vi "UHR-Fleezers Control (host) - 12.4.vi"() -> ()   [LabVIEW 2012] (continued)
                                tunnel: w627 -> [w628]
                                frame #0 {
                                n357 = property on="Trap Pos FB SP" class="DigNum (strict)"("Val(Sgnl)"=w628) -> ()  [unwired: 2 in, 2 out]
                                }
                                frame #1 {
                                n358 = Wait (ms)(milliseconds to wait=u32 700) -> ()  [unwired: 1 out]
                                }
                                frame #2 {
                                n359 = local read "Action (%)"() -> (w633:dbl)
                                n360 = Absolute Value(x=w633) -> (abs(x)=w632:dbl)
                                n361 = Greater?(x=w632, y=70.0) -> (0:w630:bool)
                                n362 = property on="Remove Action Offset" class="Bool (strict)"("Val(Sgnl)"=w630) -> ()  [unwired: 2 in, 2 out]
                                }
                                frame #3 {
                                n363 = for {
                                N: 4 -> [_]
                                n364 = flat-sequence {
                                frame #0 {
                                n365 = Wait (ms)(milliseconds to wait=u32 500) -> ()  [unwired: 1 out]
                                }
                                frame #1 {
                                n366 = local read "Action (%)"() -> (w639:dbl)
                                n367 = Absolute Value(x=w639) -> (abs(x)=w638:dbl)
                                n368 = Greater?(x=w638, y=70.0) -> (0:w636:bool)
                                n369 = property on="Remove Action Offset" class="Bool (strict)"("Val(Sgnl)"=w636) -> ()  [unwired: 2 in, 2 out]
                                }
                                }
                                }
                                }
                                frame #4 {
                                n370 = Wait (ms)(milliseconds to wait=u32 500) -> ()  [unwired: 1 out]
                                }
                                frame #5 {
                                n371 = local read "Mean"() -> (w647:dbl)
                                n372 = Greater?(x=w647, y=11.0) -> (0:w641:bool)
                                n373 = Not(x=w641) -> (.not. x?=w642:bool)
                                n374 = And(x=w642, y="Shift confocal") -> (x .and. y?=w644:bool)
                                n375 = And(x=w641, y="Shift confocal") -> (x .and. y?=w645:bool)
                                n376 = case shown="True" w645 {
                                frame False {
                                }
                                frame True {
                                n377 = local read "Confocal Y 2 (V)"() -> (w651:dbl)
                                n378 = local read "Confocal X 2 (V)"() -> (w650:dbl)
                                n379 = property on="AO1" class="Slide (strict)"("Val(Sgnl)"=w651) -> ()  [unwired: 2 in, 2 out]
                                n380 = property on="AO2" class="Slide (strict)"("Val(Sgnl)"=w650) -> ()  [unwired: 2 in, 2 out]
                                }
                                }
                                n381 = case shown="True" w644 {
                                frame False {
                                }
                                frame True {
                                n382 = local read "Confocal Y 1 (V)"() -> (w649:dbl)
                                n383 = local read "Confocal X 1 (V)"() -> (w648:dbl)
                                n384 = property on="AO1" class="Slide (strict)"("Val(Sgnl)"=w649) -> ()  [unwired: 2 in, 2 out]
                                n385 = property on="AO2" class="Slide (strict)"("Val(Sgnl)"=w648) -> ()  [unwired: 2 in, 2 out]
                                }
                                }
                                }
                                frame #6 {
                                n386 = Wait (ms)(milliseconds to wait=u32 1500) -> ()  [unwired: 1 out]
                                }
                                frame #7 {
                                n387 = property on="Rem fb disp offset" class="Bool (strict)"("Val(Sgnl)"=TRUE ("Value (Signaling)")) -> ()  [unwired: 2 in, 2 out]
                                }
                                }
                                }
                                frame True {
                                n388 = flat-sequence {
                                tunnel: w654 -> [w655]
                                frame #0 {
                                n389 = property on="Trap Delta (MHz)" class="DigNum (strict)"("Val(Sgnl)"=w655) -> ()  [unwired: 2 in, 2 out]
                                }
                                frame #1 {
                                n390 = Wait (ms)(milliseconds to wait=u32 500) -> ()  [unwired: 1 out]
                                }
                                frame #2 {
                                n391 = local read "Shift confocal"() -> (w661:bool)
                                n392 = local read "Mean"() -> (w663:dbl)
                                n393 = Greater?(x=w663, y=11.0) -> (0:w660:bool)
                                n394 = Not(x=w660) -> (.not. x?=w659:bool)
                                n395 = And(x=w659, y=w661) -> (x .and. y?=w657:bool)
                                n396 = And(x=w660, y=w661) -> (x .and. y?=w658:bool)
                                n397 = case shown="True" w658 {
                                frame False {
                                }
                                frame True {
                                n398 = local read "Confocal Y 2 (V)"() -> (w667:dbl)
                                n399 = local read "Confocal X 2 (V)"() -> (w666:dbl)
                                n400 = property on="AO2" class="Slide (strict)"("Val(Sgnl)"=w666) -> ()  [unwired: 2 in, 2 out]
                                n401 = property on="AO1" class="Slide (strict)"("Val(Sgnl)"=w667) -> ()  [unwired: 2 in, 2 out]
                                }
                                }
                                n402 = case shown="True" w657 {
                                frame False {
                                }
                                frame True {
                                n403 = local read "Confocal X 1 (V)"() -> (w664:dbl)
                                n404 = local read "Confocal Y 1 (V)"() -> (w665:dbl)
                                n405 = property on="AO2" class="Slide (strict)"("Val(Sgnl)"=w664) -> ()  [unwired: 2 in, 2 out]
                                n406 = property on="AO1" class="Slide (strict)"("Val(Sgnl)"=w665) -> ()  [unwired: 2 in, 2 out]
                                }
                                }
                                }
                                }
                                }
                                }
                                }
                                }
                                }
                                frame "Image" {
                                n407 = property on="Confocal Image" class="Bool (strict)"("Val(Sgnl)"=TRUE ("Value (Signaling)")) -> ()  [unwired: 2 in, 2 out]
                                }
                              }
                              n408 = local write "Fl. High"(FALSE ("Fl. High")) -> ()
                              n409 = local read "Time (s)"() -> (w601:dbl)
                            }
                            frame #1 {
                              n410 = case shown="True" "Auto F Reset" {
                                tunnel: w673 -> [_ w678]
                                tunnel: w672 -> [_ w677]
                                tunnel: w671 -> [_ w676]
                                tunnel: w670 -> [_ w675]
                                frame False {
                                }
                                frame True {
                                n411 = node-c288() -> (w680:T22)  [unwired: 4 in]
                                n412 = timed-loop {
                                timing: w680 -> [_]
                                timing-out: [_] -> w679
                                tunnel: w678 -> [w685]
                                tunnel: w677 -> [w684]
                                tunnel: w676 -> [w683]
                                tunnel: w675 -> [w682]
                                stop <- w681 stop-if-true
                                n413 = node-c288() -> ()  [unwired: 1 in, 1 out]
                                n414 = local read "Fl. Delta Thresh. (kHz)"() -> (w694:dbl)
                                n415 = local read "APD to Watch"() -> (w695:bool)
                                n416 = local read "Delta Fl. 1"() -> (w696:dbl)
                                n417 = local read "Delta Fl. 2"() -> (w697:dbl)
                                n418 = local read "Fl. Triggered..."() -> (w688:bool)
                                n419 = local read "Stop All"() -> (w689:bool)
                                n420 = local read "Reset Force"() -> (w687:bool)
                                n421 = Multiply(x=w694, y=1000.0) -> (x*y=w692:dbl)
                                n422 = Select(t=w696, s=w695, f=w697) -> (s? t:f=w691:dbl)
                                n423 = Not(x=w688) -> (.not. x?=w686:bool)
                                n424 = Greater?(x=w691, y=w692) -> (0:w690:bool)
                                n425 = Compound Arithmetic op=OR(w690, w689, w686, w687) -> (w681:bool)
                                n426 = case shown="True" w681 {
                                tunnel: w685 -> [_ w701]
                                tunnel: w684 -> [_ w705]
                                tunnel: w683 -> [_ w704]
                                tunnel: w682 -> [_ w703]
                                frame False {
                                }
                                frame True {
                                n427 = case shown="\"Yank\"" w705 {
                                tunnel: w704 -> [_ w715]
                                tunnel: w703 -> [_ w713]
                                frame "Image", Default {
                                }
                                frame "Yank" {
                                n428 = flat-sequence {
                                tunnel: [w718] -> w716
                                tunnel: w715 -> [w718]
                                tunnel: [w717] -> w714
                                tunnel: w713 -> [w717]
                                tunnel: w716 -> [w724]
                                tunnel: w714 -> [w722]
                                frame #0 {
                                n429 = local read "Yank Delay (s)"() -> (w721:dbl)
                                n430 = Multiply(x=w721, y=1000.0) -> (x*y=w719:dbl)
                                n431 = Wait (ms)(milliseconds to wait=w719) -> ()  [unwired: 1 out]
                                }
                                frame #1 {
                                n432 = local read "Yank to which?"() -> (w723:bool)
                                n433 = case shown="False" w723 {
                                tunnel: w724 -> [_ w752]
                                tunnel: w722 -> [w725 _]
                                frame False {
                                n434 = flat-sequence {
                                tunnel: w725 -> [w726]
                                frame #0 {
                                n435 = property on="Trap Pos FB SP" class="DigNum (strict)"("Val(Sgnl)"=w726) -> ()  [unwired: 2 in, 2 out]
                                }
                                frame #1 {
                                n436 = Wait (ms)(milliseconds to wait=u32 700) -> ()  [unwired: 1 out]
                                }
                                frame #2 {
                                n437 = local read "Action (%)"() -> (w731:dbl)
                                n438 = Absolute Value(x=w731) -> (abs(x)=w730:dbl)
                                n439 = Greater?(x=w730, y=70.0) -> (0:w728:bool)
                                n440 = property on="Remove Action Offset" class="Bool (strict)"("Val(Sgnl)"=w728) -> ()  [unwired: 2 in, 2 out]
                                }
                                frame #3 {
                                n441 = for {
                                N: 4 -> [_]
                                n442 = flat-sequence {
                                frame #0 {
                                n443 = Wait (ms)(milliseconds to wait=u32 500) -> ()  [unwired: 1 out]
                                }
                                frame #1 {
                                n444 = local read "Action (%)"() -> (w737:dbl)
                                n445 = Absolute Value(x=w737) -> (abs(x)=w736:dbl)
                                n446 = Greater?(x=w736, y=70.0) -> (0:w734:bool)
                                n447 = property on="Remove Action Offset" class="Bool (strict)"("Val(Sgnl)"=w734) -> ()  [unwired: 2 in, 2 out]
                                }
                                }
                                }
                                }
                                frame #4 {
                                n448 = Wait (ms)(milliseconds to wait=u32 500) -> ()  [unwired: 1 out]
                                }
                                frame #5 {
                                n449 = local read "Shift confocal"() -> (w742:bool)
                                n450 = local read "Mean"() -> (w745:dbl)
                                n451 = Greater?(x=w745, y=11.0) -> (0:w741:bool)
                                n452 = Not(x=w741) -> (.not. x?=w740:bool)
                                n453 = And(x=w741, y=w742) -> (x .and. y?=w743:bool)
                                n454 = And(x=w740, y=w742) -> (x .and. y?=w739:bool)
                                n455 = case shown="True" w743 {
                                frame False {
                                }
                                frame True {
                                n456 = local read "Confocal X 2 (V)"() -> (w748:dbl)
                                n457 = local read "Confocal Y 2 (V)"() -> (w749:dbl)
                                n458 = property on="AO2" class="Slide (strict)"("Val(Sgnl)"=w748) -> ()  [unwired: 2 in, 2 out]
                                n459 = property on="AO1" class="Slide (strict)"("Val(Sgnl)"=w749) -> ()  [unwired: 2 in, 2 out]
                                }
                                }
                                n460 = case shown="True" w739 {
                                frame False {
                                }
                                frame True {
                                n461 = local read "Confocal Y 1 (V)"() -> (w747:dbl)
                                n462 = local read "Confocal X 1 (V)"() -> (w746:dbl)
                                n463 = property on="AO1" class="Slide (strict)"("Val(Sgnl)"=w747) -> ()  [unwired: 2 in, 2 out]
                                n464 = property on="AO2" class="Slide (strict)"("Val(Sgnl)"=w746) -> ()  [unwired: 2 in, 2 out]
                                }
                                }
                                }
                                frame #6 {
                                n465 = Wait (ms)(milliseconds to wait=u32 1500) -> ()  [unwired: 1 out]
                                }
                                frame #7 {
                                n466 = property on="Rem fb disp offset" class="Bool (strict)"("Val(Sgnl)"=TRUE ("Value (Signaling)")) -> ()  [unwired: 2 in, 2 out]
                                }
                                }
                                }
                                frame True {
                                n467 = flat-sequence {
                                tunnel: w752 -> [w753]
                                frame #0 {
                                n468 = property on="Trap Delta (MHz)" class="DigNum (strict)"("Val(Sgnl)"=w753) -> ()  [unwired: 2 in, 2 out]
                                }
                                frame #1 {
                                n469 = Wait (ms)(milliseconds to wait=u32 500) -> ()  [unwired: 1 out]
                                }
                                frame #2 {
                                n470 = local read "Shift confocal"() -> (w759:bool)
                                n471 = local read "Mean"() -> (w760:dbl)
                                n472 = Greater?(x=w760, y=11.0) -> (0:w758:bool)
                                n473 = And(x=w758, y=w759) -> (x .and. y?=w756:bool)
                                n474 = Not(x=w758) -> (.not. x?=w757:bool)
                                n475 = And(x=w757, y=w759) -> (x .and. y?=w755:bool)
                                n476 = case shown="True" w756 {
                                frame False {
                                }
                                frame True {
                                n477 = local read "Confocal Y 2 (V)"() -> (w765:dbl)
                                n478 = local read "Confocal X 2 (V)"() -> (w764:dbl)
                                n479 = property on="AO1" class="Slide (strict)"("Val(Sgnl)"=w765) -> ()  [unwired: 2 in, 2 out]
                                n480 = property on="AO2" class="Slide (strict)"("Val(Sgnl)"=w764) -> ()  [unwired: 2 in, 2 out]
                                }
                                }
                                n481 = case shown="True" w755 {
                                frame False {
                                }
                                frame True {
                                n482 = local read "Confocal Y 1 (V)"() -> (w763:dbl)
                                n483 = local read "Confocal X 1 (V)"() -> (w762:dbl)
                                n484 = property on="AO2" class="Slide (strict)"("Val(Sgnl)"=w762) -> ()  [unwired: 2 in, 2 out]
                                n485 = property on="AO1" class="Slide (strict)"("Val(Sgnl)"=w763) -> ()  [unwired: 2 in, 2 out]
                                }
                                }
                                }
                                }
                                }
                                }
                                }
                                }
                                }
                                }
                                n486 = local read "Time (s)"() -> (w700:dbl)
                                n487 = Subtract(x=w701, y=w700) -> (x-y=w712:dbl)
                                n488 = Number To Decimal String(number=w712, width (-)=i16 0) -> (decimal integer string=w710:string)
                                n489 = Concatenate Strings(w710, " s fluorescence event") -> (w707:string)
                                n490 = local read "Messages"() -> (w708:string)
                                n491 = local write "Duration (s)"(w712) -> ()
                                n492 = call "Update messages.vi"("Message to add"=w707, "Old message string"=w708) -> ("New message string"=w706:string)
                                n493 = local write "Messages"(w706) -> ()
                                n494 = call <vilib>:"Beep.vi"() -> ()  [unwired: 12 in]
                                n495 = local write "Reset Force"(FALSE ("Force Reset")) -> ()
                                n496 = local write "Fl. High"(TRUE ("Fl. High")) -> ()
                                n497 = local write "Waiting"(TRUE ("Waiting")) -> ()
                                }
                                }
                                n498 = node-c288() -> ()  [unwired: 1 in, 1 out]
                                }
                                n499 = node-c288(w679) -> ()  [unwired: 1 out]
                                }
                              }
                            }
                          }
                          n500 = local read "Trap Delta (MHz)"() -> (w591:dbl)
                          n501 = local read "Trap Pos FB SP"() -> (w589:fxp<+/-,16,1>)
                        }
                      }
                    }
                    frame True {
                      n502 = flat-sequence {
                        tunnel: w776 -> [w786]
                        tunnel: [w786] -> w780
                        tunnel: w779 -> [w785]
                        tunnel: [w785] -> w778
                        tunnel: [w784] -> w777
                        tunnel: w775 -> [w783]
                        tunnel: [w782] -> w774
                        tunnel: w771 -> [w781]
                        tunnel: [w781] -> w770
                        tunnel: w780 -> [w856]
                        tunnel: w778 -> [w855]
                        tunnel: w777 -> [w854]
                        tunnel: w774 -> [w853]
                        tunnel: w770 -> [w852]
                        tunnel: [w853] -> w773
                        frame #0 {
                          n503 = call <vilib>:"Beep.vi"() -> ()  [unwired: 3 in, 9 out]
                          n504 = local write "Waiting"(FALSE ("Waiting")) -> ()
                          n505 = Increment(x=w783) -> (x+1=w782:u8)
                          n506 = case shown="\"Yank\"" w785 {
                            tunnel: w782 -> [_ _ w792]
                            frame "Image" {
                              n507 = property on="Confocal Image" class="Bool (strict)"("Val(Sgnl)"=TRUE ("Value (Signaling)")) -> ()  [unwired: 2 in, 2 out]
                            }
                            frame "Alarm", Default {
                            }
                            frame "Yank" {
                              n508 = flat-sequence {
                                tunnel: w792 -> [w795]
                                tunnel: [w794] -> w791
                                tunnel: ["N Array El"] -> w790
                                tunnel: w791 -> [w809]
                                tunnel: w790 -> [w805]
                                frame #0 {
                                n509 = Multiply(x="Yank Delay (s)", y=1000.0) -> (x*y=w798:dbl)
                                n510 = Quotient & Remainder(x=w795, y="N Array El") -> (x-y*floor(x/y)=w794:u8)  [unwired: 1 out]
                                n511 = Wait (ms)(milliseconds to wait=w798) -> ()  [unwired: 1 out]
                                }
                                frame #1 {
                                n512 = Random Number (0-1)() -> (number: 0 to 1=w806:dbl)
                                n513 = Multiply(x=w805, y=w806) -> (x*y=w804:dbl)
                                n514 = Round Toward -Infinity(1:w804) -> (0:w803:dbl)
                                n515 = Select(t=w803, s="Random Choice", f=w809) -> (s? t:f=w807:dbl)
                                n516 = Select(t="Yank to Trap Delta (MHz)", s="Yank to which?", f="Yank to SP") -> (s? t:f=w800:dbl[])
                                n517 = Index Array(array=w800, index=w807) -> (element=w810:dbl)
                                n518 = case shown="False" "Yank to which?" {
                                tunnel: w810 -> [w811 w837]
                                frame False {
                                n519 = flat-sequence {
                                tunnel: w811 -> [w812]
                                frame #0 {
                                n520 = property on="Trap Pos FB SP" class="DigNum (strict)"("Val(Sgnl)"=w812) -> ()  [unwired: 2 in, 2 out]
                                }
                                frame #1 {
                                n521 = Wait (ms)(milliseconds to wait=u32 700) -> ()  [unwired: 1 out]
                                }
                                frame #2 {
                                n522 = local read "Action (%)"() -> (w817:dbl)
                                n523 = Absolute Value(x=w817) -> (abs(x)=w816:dbl)
                                n524 = Greater?(x=w816, y=70.0) -> (0:w814:bool)
                                n525 = property on="Remove Action Offset" class="Bool (strict)"("Val(Sgnl)"=w814) -> ()  [unwired: 2 in, 2 out]
                                }
                                frame #3 {
                                n526 = for {
                                N: 4 -> [_]
                                n527 = flat-sequence {
                                frame #0 {
                                n528 = Wait (ms)(milliseconds to wait=u32 500) -> ()  [unwired: 1 out]
                                }
                                frame #1 {
                                n529 = local read "Action (%)"() -> (w823:dbl)
                                n530 = Absolute Value(x=w823) -> (abs(x)=w822:dbl)
                                n531 = Greater?(x=w822, y=70.0) -> (0:w820:bool)
                                n532 = property on="Remove Action Offset" class="Bool (strict)"("Val(Sgnl)"=w820) -> ()  [unwired: 2 in, 2 out]
                                }
                                }
                                }
                                }
                                frame #4 {
                                n533 = local read "Shift confocal"() -> (w827:bool)
                                n534 = local read "Mean"() -> (w830:dbl)
                                n535 = Greater?(x=w830, y=11.0) -> (0:w826:bool)
                                n536 = Not(x=w826) -> (.not. x?=w825:bool)
                                n537 = And(x=w825, y=w827) -> (x .and. y?=w824:bool)
                                n538 = And(x=w826, y=w827) -> (x .and. y?=w828:bool)
                                n539 = case shown="True" w828 {
                                frame False {
                                }
                                frame True {
                                n540 = local read "Confocal X 2 (V)"() -> (w833:dbl)
                                n541 = local read "Confocal Y 2 (V)"() -> (w834:dbl)
                                n542 = property on="AO2" class="Slide (strict)"("Val(Sgnl)"=w833) -> ()  [unwired: 2 in, 2 out]
                                n543 = property on="AO1" class="Slide (strict)"("Val(Sgnl)"=w834) -> ()  [unwired: 2 in, 2 out]
                                }
                                }
                                n544 = case shown="True" w824 {
                                frame False {
                                }
                                frame True {
                                n545 = local read "Confocal X 1 (V)"() -> (w831:dbl)
                                n546 = local read "Confocal Y 1 (V)"() -> (w832:dbl)
                                n547 = property on="AO1" class="Slide (strict)"("Val(Sgnl)"=w832) -> ()  [unwired: 2 in, 2 out]
                                n548 = property on="AO2" class="Slide (strict)"("Val(Sgnl)"=w831) -> ()  [unwired: 2 in, 2 out]
                                }
                                }
                                }
                                frame #5 {
                                n549 = Wait (ms)(milliseconds to wait=u32 1500) -> ()  [unwired: 1 out]
                                }
                                frame #6 {
                                n550 = property on="Rem fb disp offset" class="Bool (strict)"("Val(Sgnl)"=TRUE ("Value (Signaling)")) -> ()  [unwired: 2 in, 2 out]
                                }
                                }
                                }
                                frame True {
                                n551 = flat-sequence {
                                tunnel: w837 -> [w838]
                                frame #0 {
                                n552 = property on="Trap Delta (MHz)" class="DigNum (strict)"("Val(Sgnl)"=w838) -> ()  [unwired: 2 in, 2 out]
                                }
                                frame #1 {
                                n553 = Wait (ms)(milliseconds to wait=u32 500) -> ()  [unwired: 1 out]
                                }
                                frame #2 {
                                n554 = local read "Shift confocal"() -> (w842:bool)
                                n555 = local read "Mean"() -> (w840:dbl)
                                n556 = Greater?(x=w840, y=11.0) -> (0:w843:bool)
                                n557 = Not(x=w843) -> (.not. x?=w844:bool)
                                n558 = And(x=w844, y=w842) -> (x .and. y?=w846:bool)
                                n559 = And(x=w843, y=w842) -> (x .and. y?=w845:bool)
                                n560 = case shown="True" w845 {
                                frame False {
                                }
                                frame True {
                                n561 = local read "Confocal Y 2 (V)"() -> (w850:dbl)
                                n562 = local read "Confocal X 2 (V)"() -> (w849:dbl)
                                n563 = property on="AO1" class="Slide (strict)"("Val(Sgnl)"=w850) -> ()  [unwired: 2 in, 2 out]
                                n564 = property on="AO2" class="Slide (strict)"("Val(Sgnl)"=w849) -> ()  [unwired: 2 in, 2 out]
                                }
                                }
                                n565 = case shown="True" w846 {
                                frame False {
                                }
                                frame True {
                                n566 = local read "Confocal X 1 (V)"() -> (w847:dbl)
                                n567 = local read "Confocal Y 1 (V)"() -> (w848:dbl)
                                n568 = property on="AO2" class="Slide (strict)"("Val(Sgnl)"=w847) -> ()  [unwired: 2 in, 2 out]
                                n569 = property on="AO1" class="Slide (strict)"("Val(Sgnl)"=w848) -> ()  [unwired: 2 in, 2 out]
                                }
                                }
                                }
                                }
                                }
                                }
                                }
                              }
                            }
                          }
                          n570 = local read "Time (s)"() -> (w784:dbl)
                          "Fl. High" <- TRUE ("Yanking")
                        }
                        frame #1 {
                          n571 = local read "Auto F Reset"() -> (w851:bool)
                          n572 = case shown="True" w851 {
                            tunnel: w856 -> [_ w860]
                            tunnel: w855 -> [_ w859]
                            tunnel: w854 -> [_ w858]
                            tunnel: w852 -> [_ w857]
                            frame False {
                            }
                            frame True {
                              n573 = node-c288() -> (w862:T22)  [unwired: 4 out]
                              n574 = timed-loop {
                                timing: w862 -> [_]
                                timing-out: [_] -> w861
                                tunnel: w860 -> [w880]
                                tunnel: w859 -> [w879]
                                tunnel: w858 -> [w878]
                                tunnel: w857 -> [w877]
                                stop <- w863 stop-if-true
                                n575 = node-c288() -> ()  [unwired: 2 out]
                                n576 = local read "Fl. Delta Thresh. (kHz)"() -> (w871:dbl)
                                n577 = local read "Fl. Triggered..."() -> (w876:bool)
                                n578 = local read "Delta Fl. 1"() -> (w867:dbl)
                                n579 = local read "Delta Fl. 2"() -> (w865:dbl)
                                n580 = local read "Stop All"() -> (w874:bool)
                                n581 = local read "APD to Watch"() -> (w866:bool)
                                n582 = Select(t=w867, s=w866, f=w865) -> (s? t:f=w864:dbl)
                                n583 = Not(x=w876) -> (.not. x?=w875:bool)
                                n584 = Multiply(x=w871, y=1000.0) -> (x*y=w870:dbl)
                                n585 = Negate(x=w870) -> (-x=w869:dbl)
                                n586 = Less?(x=w864, y=w869) -> (x < y?=w873:bool)
                                n587 = Compound Arithmetic op=OR(w873, w874, w875, "Reset Force") -> (w863:bool)
                                n588 = case shown="True" w863 {
                                tunnel: w880 -> [_ w895]
                                tunnel: w879 -> [_ w894]
                                tunnel: w878 -> [_ w884]
                                tunnel: w877 -> [_ w886]
                                frame False {
                                }
                                frame True {
                                n589 = local read "Time (s)"() -> (w885:dbl)
                                n590 = case shown="\"Yank\"" w894 {
                                tunnel: w895 -> [_ w898]
                                tunnel: w886 -> [_ w896]
                                frame "Image", Default {
                                }
                                frame "Yank" {
                                n591 = flat-sequence {
                                tunnel: [w904] -> w899
                                tunnel: w898 -> [w904]
                                tunnel: [w900] -> w897
                                tunnel: w896 -> [w900]
                                tunnel: w899 -> [w907]
                                tunnel: w897 -> [w905]
                                frame #0 {
                                n592 = local read "Yank Delay (s)"() -> (w903:dbl)
                                n593 = Multiply(x=w903, y=1000.0) -> (x*y=w901:dbl)
                                n594 = Wait (ms)(milliseconds to wait=w901) -> ()  [unwired: 1 out]
                                }
                                frame #1 {
                                n595 = local read "Yank to which?"() -> (w906:bool)
                                n596 = case shown="False" w906 {
                                tunnel: w907 -> [_ w934]
                                tunnel: w905 -> [w908 _]
                                frame False {
                                n597 = flat-sequence {
                                tunnel: w908 -> [w909]
                                frame #0 {
                                n598 = property on="Trap Pos FB SP" class="DigNum (strict)"("Val(Sgnl)"=w909) -> ()  [unwired: 2 in, 2 out]
                                }
                                frame #1 {
                                n599 = Wait (ms)(milliseconds to wait=u32 700) -> ()  [unwired: 1 out]
                                }
                                frame #2 {
                                n600 = local read "Action (%)"() -> (w914:dbl)
                                n601 = Absolute Value(x=w914) -> (abs(x)=w913:dbl)
                                n602 = Greater?(x=w913, y=70.0) -> (0:w911:bool)
                                n603 = property on="Remove Action Offset" class="Bool (strict)"("Val(Sgnl)"=w911) -> ()  [unwired: 2 in, 2 out]
                                }
                                frame #3 {
                                n604 = for {
                                N: 4 -> [_]
                                n605 = flat-sequence {
                                frame #0 {
                                n606 = Wait (ms)(milliseconds to wait=u32 500) -> ()  [unwired: 1 out]
                                }
                                frame #1 {
                                n607 = local read "Action (%)"() -> (w920:dbl)
                                n608 = Absolute Value(x=w920) -> (abs(x)=w919:dbl)
                                n609 = Greater?(x=w919, y=70.0) -> (0:w917:bool)
                                n610 = property on="Remove Action Offset" class="Bool (strict)"("Val(Sgnl)"=w917) -> ()  [unwired: 2 in, 2 out]
                                }
                                }
                                }
                                }
                                frame #4 {
                                n611 = local read "Shift confocal"() -> (w925:bool)
                                n612 = local read "Mean"() -> (w927:dbl)
                                n613 = Greater?(x=w927, y=11.0) -> (0:w924:bool)
                                n614 = Not(x=w924) -> (.not. x?=w923:bool)
                                n615 = And(x=w924, y=w925) -> (x .and. y?=w922:bool)
                                n616 = And(x=w923, y=w925) -> (x .and. y?=w921:bool)
                                n617 = case shown="True" w922 {
                                frame False {
                                }
                                frame True {
                                n618 = local read "Confocal Y 2 (V)"() -> (w931:dbl)
                                n619 = local read "Confocal X 2 (V)"() -> (w930:dbl)
                                n620 = property on="AO2" class="Slide (strict)"("Val(Sgnl)"=w930) -> ()  [unwired: 2 in, 2 out]
                                n621 = property on="AO1" class="Slide (strict)"("Val(Sgnl)"=w931) -> ()  [unwired: 2 in, 2 out]
                                }
                                }
                                n622 = case shown="True" w921 {
                                frame False {
                                }
                                frame True {
                                n623 = local read "Confocal X 1 (V)"() -> (w928:dbl)
                                n624 = local read "Confocal Y 1 (V)"() -> (w929:dbl)
                                n625 = property on="AO1" class="Slide (strict)"("Val(Sgnl)"=w929) -> ()  [unwired: 2 in, 2 out]
                                n626 = property on="AO2" class="Slide (strict)"("Val(Sgnl)"=w928) -> ()  [unwired: 2 in, 2 out]
                                }
                                }
                                }
                                frame #5 {
                                n627 = Wait (ms)(milliseconds to wait=u32 1500) -> ()  [unwired: 1 out]
                                }
                                frame #6 {
                                n628 = property on="Rem fb disp offset" class="Bool (strict)"("Val(Sgnl)"=TRUE ("Value (Signaling)")) -> ()  [unwired: 2 in, 2 out]
                                }
                                }
                                }
                                frame True {
                                n629 = flat-sequence {
                                tunnel: w934 -> [w935]
                                frame #0 {
                                n630 = property on="Trap Delta (MHz)" class="DigNum (strict)"("Val(Sgnl)"=w935) -> ()  [unwired: 2 in, 2 out]
                                }
                                frame #1 {
                                n631 = Wait (ms)(milliseconds to wait=u32 500) -> ()  [unwired: 1 out]
                                }
                                frame #2 {
                                n632 = local read "Shift confocal"() -> (w941:bool)
                                n633 = local read "Mean"() -> (w943:dbl)
                                n634 = Greater?(x=w943, y=11.0) -> (0:w940:bool)
                                n635 = Not(x=w940) -> (.not. x?=w939:bool)
                                n636 = And(x=w940, y=w941) -> (x .and. y?=w938:bool)
                                n637 = And(x=w939, y=w941) -> (x .and. y?=w937:bool)
                                n638 = case shown="True" w938 {
                                frame False {
                                }
                                frame True {
                                n639 = local read "Confocal Y 2 (V)"() -> (w947:dbl)
                                n640 = local read "Confocal X 2 (V)"() -> (w946:dbl)
                                n641 = property on="AO2" class="Slide (strict)"("Val(Sgnl)"=w946) -> ()  [unwired: 2 in, 2 out]
                                n642 = property on="AO1" class="Slide (strict)"("Val(Sgnl)"=w947) -> ()  [unwired: 2 in, 2 out]
                                }
                                }
                                n643 = case shown="True" w937 {
                                frame False {
                                }
                                frame True {
                                n644 = local read "Confocal Y 1 (V)"() -> (w945:dbl)
                                n645 = local read "Confocal X 1 (V)"() -> (w944:dbl)
                                n646 = property on="AO2" class="Slide (strict)"("Val(Sgnl)"=w944) -> ()  [unwired: 2 in, 2 out]
                                n647 = property on="AO1" class="Slide (strict)"("Val(Sgnl)"=w945) -> ()  [unwired: 2 in, 2 out]
                                }
                                }
                                }
                                }
                                }
                                }
                                }
                                }
                                }
                                }
                                n648 = local read "Messages"() -> (w893:string)
                                n649 = Subtract(x=w885, y=w884) -> (x-y=w891:dbl)
                                "Duration (s)" <- w891
                                n650 = Number To Decimal String(number=w891, width (-)=i16 0) -> (decimal integer string=w889:string)
                                n651 = Concatenate Strings(w889, " s fluorescence event." ("string")) -> (w887:string)
                                n652 = call "Update messages.vi"("Message to add"=w887, "Old message string"=w893) -> ("New message string"=w892:string)
                                n653 = local write "Reset Force"(FALSE ("Reset Force")) -> ()
                                n654 = local write "Waiting"(TRUE ("Waiting")) -> ()
                                n655 = local write "Messages"(w892) -> ()
                                n656 = local write "Fl. High"(FALSE ("Fl. High")) -> ()
                                n657 = call <vilib>:"Beep.vi"() -> ()  [unwired: 3 in, 9 out]
                                }
                                }
                                n658 = node-c288() -> ()  [unwired: 2 out]
                              }
                              n659 = node-c288(w861) -> ()  [unwired: 1 out]
                            }
                          }
                        }
                      }
                      n660 = local read "Trap Delta (MHz)"() -> (w776:dbl)
                      n661 = local read "Trap Pos FB SP"() -> (w771:fxp<+/-,16,1>)
                    }
                  }
                }
                frame #1 {
                  n662 = local read "Stop All"() -> (w957:bool)
                  n663 = local read "Fl. Triggered..."() -> (w955:bool)
                  n664 = Not(x=w955) -> (.not. x?=w956:bool)
                  n665 = Or(x=w956, y=w957) -> (x .or. y?=w954:bool)
                }
              }
              n666 = case shown="True" w548 {
                frame False {
                }
                frame True {
                  n667 = local read "Confocal Y 1 (V)"() -> (w558:dbl)
                  n668 = local read "Confocal X 1 (V)"() -> (w557:dbl)
                  n669 = property on="AO2" class="Slide (strict)"("Val(Sgnl)"=w557) -> ()  [unwired: 2 in, 2 out]
                  n670 = property on="AO1" class="Slide (strict)"("Val(Sgnl)"=w558) -> ()  [unwired: 2 in, 2 out]
                }
              }
              n671 = case shown="True" w548 {
                frame False {
                }
                frame True {
                  w556 = FALSE ("Fl. High")
                  n672 = local write "Waiting"(w556) -> ()
                  n673 = local write "Fl. High"(w556) -> ()
                }
              }
              n674 = node-c288() -> ()  [unwired: 2 out]
            }
            n675 = node-c288(w546) -> ()  [unwired: 1 out]
          }
        }
      }
      event "Stop All": Value Change {
        n676 = event-data() -> ()  [unwired: 7 out]
        n677 = local read "Stop All"() -> (w962:bool)
      }
    }
    n678 = node-c288() -> ()  [unwired: 2 out]
  }
  n679 = timed-loop "Run Scripts, including: stage motion" {
    tunnel: w119 -> [w970]
    tunnel: w118 -> [w971]
    tunnel: [w971] -> w117
    tunnel: [w970] -> w116
    timing: w114 -> [_]
    timing-out: [_] -> w113
    tunnel: w100 -> [w969]
    tunnel: w101 -> [w968]
    tunnel: w72 -> [w965]
    tunnel: w71 -> [w964]
    tunnel: w70 -> [w966]
    tunnel: w69 -> [w967]
    tunnel: w2 -> [w963]
    stop <- w972 stop-if-true
    n680 = node-c288() -> ()  [unwired: 1 in, 1 out]
    n681 = event shown="[20] \"Stop All\": Value Change" {
      selector: _ -> [_ _ _ _ _ _ _ _ _ _ _ _ _ _ _ _ _ _ _ _ _]
      dyn-events: _ -> [_ _ _ _ _ _ _ _ _ _ _ _ _ _ _ _ _ _ _ _ _]
      timeout: _ -> [_ _ _ _ _ _ _ _ _ _ _ _ _ _ _ _ _ _ _ _ _]
      tunnel: ["Set Position" "Move to Position" _ _ _ _ "Read Harvard" _ _ _ _ _ _ "Got ADig bead" "Force FB Data\nScript" _ "Got DNA bead" "Take Stepping Data" _ "Take Detection Laser\nImage" _] -> _
      tunnel: [_ _ _ _ _ _ _ _ _ _ _ _ _ _ _ _ _ _ _ _ w1624] -> w972
      tunnel: w970 -> [w990 w998 w1011 w1041 _ _ _ w1115 w1155 w1236 w1265 w1397 w1423 _ w1459 _ _ _ _ _ _]
      tunnel: w971 -> [w991 w999 w1012 w1042 _ _ _ w1116 w1156 w1237 w1266 w1398 w1424 _ w1460 _ _ _ _ _ _]
      tunnel: w969 -> [_ _ _ _ _ _ w1100 _ _ _ _ _ _ _ _ _ _ _ _ _ _]
      tunnel: w968 -> [_ _ _ _ _ _ w1099 _ _ _ _ _ _ _ _ _ _ _ _ _ _]
      tunnel: w967 -> [_ _ _ _ _ _ _ _ _ _ _ _ _ _ _ _ _ _ _ _ _]
      tunnel: w966 -> [_ _ _ _ _ _ _ _ _ _ _ _ _ _ _ _ _ _ _ _ _]
      tunnel: w965 -> [_ _ _ _ _ _ _ _ _ _ _ _ _ _ _ _ _ _ _ _ _]
      tunnel: w964 -> [_ _ _ _ _ _ _ _ _ _ _ _ _ _ _ _ _ _ _ _ _]
      tunnel: w963 -> [_ _ _ _ w1069 w1090 _ _ _ _ _ _ _ _ _ _ _ _ _ _ w1623]
      event "Set Position", "Set Position 2", "Set Position 3", "Set Position 4", "Set Position 5", "Set Position 1": Value Change {
        n682 = event-data() -> ()  [unwired: 1 in, 5 out]
        n683 = Build Array("Set Position 1", "Set Position 2", "Set Position 3", "Set Position 4", "Set Position 5") -> (w989:bool[])
        n684 = Boolean Array To Number(Boolean array=w989) -> (number=w988:u32)
        n685 = Logarithm Base 2(1:w988) -> (0:w980:dbl)
        n686 = call "Read Stage Position.vi"("error in"=w990, "VISA resource name in"=w991) -> ("Current Position"=w995:cluster{dbl, dbl, dbl}, "error out"=w994:errorcluster)  [unwired: 2 out]
        n687 = Decrement(x="Position") -> (x-1=w978:dbl)
        n688 = Greater Or Equal?(x=w980, y=0.0) -> (x >= y?=w981:bool)
        n689 = Cluster To Array(cluster=w995) -> (array=w992:dbl[])
        n690 = local write "Stage Control Serial Error"(w994) -> ()
        n691 = Select(t=w980, s=w981, f=w978) -> (s? t:f=w977:dbl)
        n692 = Increment(x=w977) -> (x+1=w976:dbl)
        n693 = Build Array (concatenate)(w976, w992) -> (w975:dbl[])
        n694 = Replace Array Subset(array="Saved Stage Positions", new element=w975, index (row)=w977) -> (w993:dbl[][])  [unwired: 1 in]
        n695 = local write "Saved Stage Positions"(w993) -> ()
      }
      event "Move to Position": Value Change {
        n696 = event-data() -> ()  [unwired: 1 in, 5 out]
        n697 = flat-sequence {
          tunnel: w999 -> [w1003]
          tunnel: w998 -> [w1002]
          frame #0 {
            n698 = local read "Saved Stage Positions"() -> (w1005:dbl[][])
            n699 = local read "Position"() -> (w1004:dbl)
            n700 = local write "Stage Moving"(TRUE ("Stage Moving")) -> ()
            n701 = call "move to saved stage position.vi"("error in"=w1002, "Stage VISA resource name in"=w1003, "Position"=w1004, "Saved Stage Positions"=w1005) -> ("error out"=w1001:errorcluster)  [unwired: 1 out]
            n702 = local write "Stage Control Serial Error"(w1001) -> ()
          }
          frame #1 {
            n703 = call <vilib>:"Beep.vi"() -> ()  [unwired: 3 in, 9 out]
            n704 = local write "Stage Moving"(FALSE ("Stage Moving")) -> ()
          }
        }
      }
      event "Move Cap. 1 (DNA Bottom)": Value Change {
        n705 = event-data() -> ()  [unwired: 1 in, 5 out]
        n706 = local write "Move Cap. 1 (DNA Bottom)"(FALSE ("Move Cap. 1 (DNA Right)")) -> ()
        n707 = flat-sequence {
          tunnel: w1011 -> [w1014]
          tunnel: w1012 -> [w1015]
          tunnel: [w1015] -> w1009
          tunnel: [w1014] -> w1008
          tunnel: w1009 -> [w1017]
          tunnel: w1008 -> [w1016]
          frame #0 {
            n708 = property on="Sample Channel\nFlow" class="Bool (strict)"("Val(Sgnl)"="Cap 1 Samp Flow ON") -> ()  [unwired: 2 in, 2 out]
          }
          frame #1 {
            n709 = local read "Saved Stage Positions"() -> (w1027:dbl[][])
            n710 = local write "Stage Moving"(TRUE ("Stage Moving")) -> ()
            n711 = Array Subset(array=w1027, index (row)=0 ("index"), length (row)=1 ("length"), index (col)=1 ("index"), length (col)=3 ("length")) -> (w1024:dbl[][])
            n712 = Reshape Array(w1024, 3 ("dimension size")) -> (w1022:dbl[])
            n713 = Array To Cluster(array=w1022) -> (cluster=w1021:cluster{"[0]":dbl, "[1]":dbl, "[2]":dbl})
            n714 = call "Set Stage Position.vi"("Position"=w1021, "error in"=w1016, "VISA resource name in"=w1017) -> ("error out"=w1020:errorcluster)  [unwired: 2 out]
            n715 = local write "Stage Control Serial Error"(w1020) -> ()
          }
          frame #2 {
            n716 = local write "Stage Moving"(FALSE ("Stage Moving")) -> ()
            n717 = case shown="True" "Cap 1 Flow ON" {
              frame False {
              }
              frame True {
                n718 = property on="Inject Pump 1" class="Bool (strict)"("Val(Sgnl)"=TRUE ("Value (Signaling)")) -> ()  [unwired: 2 in, 2 out]
              }
            }
            n719 = call <vilib>:"Beep.vi"() -> ()  [unwired: 3 in, 9 out]
          }
          frame #3 {
            n720 = property on="Sample Channel\nFlow" class="Bool (strict)"("Val(Sgnl)"=FALSE ("Value (Signaling)")) -> ()  [unwired: 2 in, 2 out]
            n721 = local read "Cap. 2 BD T1?\n(ADig T1, DNA T2)"() -> (w1034:bool)
            n722 = case shown="True" w1034 {
              tunnel: "Cap 1 T ON" -> [w1036 w1037]
              frame False {
                n723 = property on="Trap 1 (ON/OFF)" class="Bool (strict)"("Val(Sgnl)"=w1036) -> ()  [unwired: 2 in, 2 out]
              }
              frame True {
                n724 = property on="Trap 2 (ON/OFF)" class="Bool (strict)"("Val(Sgnl)"=w1037) -> ()  [unwired: 2 in, 2 out]
              }
            }
            n725 = property on="Got DNA bead" class="Bool"("Key Focus"=TRUE) -> ()  [unwired: 2 in, 2 out]
          }
        }
      }
      event "Move Cap. 2 (ADig Top)": Value Change {
        n726 = event-data() -> ()  [unwired: 1 in, 5 out]
        n727 = local write "Move Cap. 2 (ADig Top)"(FALSE ("Move Cap. 2 (ADig Left)")) -> ()
        n728 = flat-sequence {
          tunnel: w1041 -> [w1044]
          tunnel: w1042 -> [w1045]
          tunnel: [w1045] -> w1039
          tunnel: [w1044] -> w1038
          tunnel: w1039 -> [w1048]
          tunnel: w1038 -> [w1047]
          frame #0 {
            n729 = property on="Sample Channel\nFlow" class="Bool (strict)"("Val(Sgnl)"="Cap 2 Samp Flow ON") -> ()  [unwired: 2 in, 2 out]
          }
          frame #1 {
            w1046 = FALSE ("Value (Signaling)")
            n730 = local read "Saved Stage Positions"() -> (w1058:dbl[][])
            n731 = local write "Stage Moving"(TRUE ("Stage Moving")) -> ()
            n732 = Array Subset(array=w1058, index (row)=1 ("index"), length (row)=1 ("length"), index (col)=1 ("index"), length (col)=3 ("length")) -> (w1055:dbl[][])
            n733 = Reshape Array(w1055, 3 ("dimension size")) -> (w1053:dbl[])
            n734 = property on="Trap 1 (ON/OFF)" class="Bool (strict)"("Val(Sgnl)"=w1046) -> ()  [unwired: 2 in, 2 out]